vi "FlexMag - 23-03-2023.vi"() -> ()   [LabVIEW 2018] (continued)
                                }
                                }
                                }
                                }
                                }
                                }
                                }
                                }
                                frame True {
                                }
                                }
                                }
                                frame #6 {
                                n21201 = local read "abort ch3"() -> (w25287:bool)
                                n21202 = case shown="False" w25287 {
                                frame False {
                                n21203 = local read "coating start"() -> (w25288:bool)
                                n21204 = case shown="True" w25288 {
                                frame False {
                                }
                                frame True {
                                n21205 = local read "R dc step length 7"() -> (w25291:dbl)
                                n21206 = Greater?(x=w25291, y=0.0) -> (0:w25290:bool)
                                n21207 = case shown="True" w25290 {
                                frame False {
                                }
                                frame True {
                                n21208 = flat-sequence {
                                frame #0 {
                                n21209 = local read "R dc step length 7"() -> (w25298:dbl)
                                n21210 = local read "R dc step power 7"() -> (w25293:dbl)
                                n21211 = local read "R web speed"() -> (w25297:dbl)
                                n21212 = Divide(x=w25298, y=w25297) -> (x/y=w25296:dbl)
                                n21213 = Wait (ms)(milliseconds to wait=u32 100) -> ()  [unwired: 1 out]
                                n21214 = local write "Set DC Power ch2"(w25293) -> ()
                                n21215 = Multiply(x=w25296, y=60) -> (x*y=w25294:dbl)
                                n21216 = local write "time counting"(w25294) -> ()
                                }
                                frame #1 {
                                n21217 = local write "Dc_auto_set"(TRUE ("Dc_auto_set")) -> ()
                                }
                                frame #2 {
                                n21218 = while {
                                stop <- w25301 stop-if-true
                                n21219 = local read "time counting"() -> (w25307:dbl)
                                n21220 = local read "coating start"() -> (w25305:bool)
                                n21221 = local read "abort ch3"() -> (w25303:bool)
                                n21222 = Wait Until Next ms Multiple(millisecond multiple=u32 1000) -> ()  [unwired: 1 out]
                                n21223 = Decrement(x=w25307) -> (x-1=w25306:dbl)
                                n21224 = local write "time counting"(w25306) -> ()
                                n21225 = Not(x=w25305) -> (.not. x?=w25304:bool)
                                n21226 = Less Or Equal To 0?(x=w25306) -> (x <= 0?=w25302:bool)
                                n21227 = Compound Arithmetic op=OR(w25302, w25304, w25303) -> (w25301:bool)
                                }
                                }
                                }
                                }
                                }
                                }
                                }
                                }
                                frame True {
                                }
                                }
                                }
                                frame #7 {
                                n21228 = local read "abort ch3"() -> (w25308:bool)
                                n21229 = case shown="False" w25308 {
                                frame False {
                                n21230 = local read "coating start"() -> (w25309:bool)
                                n21231 = case shown="True" w25309 {
                                frame False {
                                }
                                frame True {
                                n21232 = local read "R dc step length 8"() -> (w25312:dbl)
                                n21233 = Greater?(x=w25312, y=0.0) -> (0:w25311:bool)
                                n21234 = case shown="True" w25311 {
                                frame False {
                                }
                                frame True {
                                n21235 = flat-sequence {
                                frame #0 {
                                n21236 = local read "R dc step length 8"() -> (w25319:dbl)
                                n21237 = local read "R dc step power 8"() -> (w25314:dbl)
                                n21238 = local read "R web speed"() -> (w25318:dbl)
                                n21239 = Wait (ms)(milliseconds to wait=u32 100) -> ()  [unwired: 1 out]
                                n21240 = Divide(x=w25319, y=w25318) -> (x/y=w25317:dbl)
                                n21241 = local write "Set DC Power ch2"(w25314) -> ()
                                n21242 = Multiply(x=w25317, y=60) -> (x*y=w25315:dbl)
                                n21243 = local write "time counting"(w25315) -> ()
                                }
                                frame #1 {
                                n21244 = local write "Dc_auto_set"(TRUE ("Dc_auto_set")) -> ()
                                }
                                frame #2 {
                                n21245 = while {
                                stop <- w25322 stop-if-true
                                n21246 = local read "time counting"() -> (w25328:dbl)
                                n21247 = local read "coating start"() -> (w25326:bool)
                                n21248 = Wait Until Next ms Multiple(millisecond multiple=u32 1000) -> ()  [unwired: 1 out]
                                n21249 = local read "abort ch3"() -> (w25324:bool)
                                n21250 = Decrement(x=w25328) -> (x-1=w25327:dbl)
                                n21251 = local write "time counting"(w25327) -> ()
                                n21252 = Not(x=w25326) -> (.not. x?=w25325:bool)
                                n21253 = Less Or Equal To 0?(x=w25327) -> (x <= 0?=w25323:bool)
                                n21254 = Compound Arithmetic op=OR(w25323, w25325, w25324) -> (w25322:bool)
                                }
                                }
                                }
                                }
                                }
                                }
                                }
                                }
                                frame True {
                                }
                                }
                                }
                                frame #8 {
                                n21255 = local read "abort ch3"() -> (w25329:bool)
                                n21256 = case shown="False" w25329 {
                                frame False {
                                n21257 = local read "coating start"() -> (w25330:bool)
                                n21258 = case shown="True" w25330 {
                                frame False {
                                }
                                frame True {
                                n21259 = local read "R dc step length 9"() -> (w25333:dbl)
                                n21260 = Greater?(x=w25333, y=0.0) -> (0:w25332:bool)
                                n21261 = case shown="True" w25332 {
                                frame False {
                                }
                                frame True {
                                n21262 = flat-sequence {
                                frame #0 {
                                n21263 = local read "R dc step length 9"() -> (w25340:dbl)
                                n21264 = local read "R dc step power 9"() -> (w25335:dbl)
                                n21265 = local read "R web speed"() -> (w25339:dbl)
                                n21266 = Wait (ms)(milliseconds to wait=u32 100) -> ()  [unwired: 1 out]
                                n21267 = Divide(x=w25340, y=w25339) -> (x/y=w25338:dbl)
                                n21268 = local write "Set DC Power ch2"(w25335) -> ()
                                n21269 = Multiply(x=w25338, y=60) -> (x*y=w25336:dbl)
                                n21270 = local write "time counting"(w25336) -> ()
                                }
                                frame #1 {
                                n21271 = local write "Dc_auto_set"(TRUE ("Dc_auto_set")) -> ()
                                }
                                frame #2 {
                                n21272 = while {
                                stop <- w25343 stop-if-true
                                n21273 = local read "time counting"() -> (w25349:dbl)
                                n21274 = local read "coating start"() -> (w25347:bool)
                                n21275 = local read "abort ch3"() -> (w25345:bool)
                                n21276 = Wait Until Next ms Multiple(millisecond multiple=u32 1000) -> ()  [unwired: 1 out]
                                n21277 = Decrement(x=w25349) -> (x-1=w25348:dbl)
                                n21278 = local write "time counting"(w25348) -> ()
                                n21279 = Not(x=w25347) -> (.not. x?=w25346:bool)
                                n21280 = Less Or Equal To 0?(x=w25348) -> (x <= 0?=w25344:bool)
                                n21281 = Compound Arithmetic op=OR(w25344, w25346, w25345) -> (w25343:bool)
                                }
                                }
                                }
                                }
                                }
                                }
                                }
                                }
                                frame True {
                                }
                                }
                                }
                                frame #9 {
                                n21282 = local read "abort ch3"() -> (w25350:bool)
                                n21283 = case shown="False" w25350 {
                                frame False {
                                n21284 = local read "coating start"() -> (w25351:bool)
                                n21285 = case shown="True" w25351 {
                                frame False {
                                }
                                frame True {
                                n21286 = local read "R dc step length 10"() -> (w25354:dbl)
                                n21287 = Greater?(x=w25354, y=0.0) -> (0:w25353:bool)
                                n21288 = case shown="True" w25353 {
                                frame False {
                                }
                                frame True {
                                n21289 = flat-sequence {
                                frame #0 {
                                n21290 = local read "R dc step length 10"() -> (w25361:dbl)
                                n21291 = local read "R dc step power 10"() -> (w25356:dbl)
                                n21292 = local read "R web speed"() -> (w25360:dbl)
                                n21293 = Divide(x=w25361, y=w25360) -> (x/y=w25359:dbl)
                                n21294 = local write "Set DC Power ch2"(w25356) -> ()
                                n21295 = Wait (ms)(milliseconds to wait=u32 100) -> ()  [unwired: 1 out]
                                n21296 = Multiply(x=w25359, y=60) -> (x*y=w25357:dbl)
                                n21297 = local write "time counting"(w25357) -> ()
                                }
                                frame #1 {
                                n21298 = local write "Dc_auto_set"(TRUE ("Dc_auto_set")) -> ()
                                }
                                frame #2 {
                                n21299 = while {
                                stop <- w25364 stop-if-true
                                n21300 = local read "time counting"() -> (w25370:dbl)
                                n21301 = local read "coating start"() -> (w25368:bool)
                                n21302 = local read "abort ch3"() -> (w25366:bool)
                                n21303 = Wait Until Next ms Multiple(millisecond multiple=u32 1000) -> ()  [unwired: 1 out]
                                n21304 = Decrement(x=w25370) -> (x-1=w25369:dbl)
                                n21305 = local write "time counting"(w25369) -> ()
                                n21306 = Not(x=w25368) -> (.not. x?=w25367:bool)
                                n21307 = Less Or Equal To 0?(x=w25369) -> (x <= 0?=w25365:bool)
                                n21308 = Compound Arithmetic op=OR(w25365, w25367, w25366) -> (w25364:bool)
                                }
                                }
                                }
                                }
                                }
                                }
                                }
                                }
                                frame True {
                                }
                                }
                                }
                                frame #10 {
                                n21309 = local read "abort ch3"() -> (w25371:bool)
                                n21310 = case shown="False" w25371 {
                                frame False {
                                n21311 = local read "coating start"() -> (w25372:bool)
                                n21312 = case shown="True" w25372 {
                                frame False {
                                }
                                frame True {
                                n21313 = Wait (ms)(milliseconds to wait=u32 100) -> ()  [unwired: 1 out]
                                "coating ch3 led 12" <- TRUE ("coating ch2 led 1")
                                }
                                }
                                }
                                frame True {
                                }
                                }
                                }
                                }
                                }
                                frame Enabled {
                                n21314 = stacked-sequence {
                                frame #0 {
                                n21315 = local read "abort ch3"() -> (w25375:bool)
                                n21316 = case shown="False" w25375 {
                                frame False {
                                n21317 = local read "coating start"() -> (w25376:bool)
                                n21318 = case shown="True" w25376 {
                                frame False {
                                }
                                frame True {
                                n21319 = local read "dep. for?"() -> (w25377:bool)
                                n21320 = case shown="False" w25377 {
                                frame False {
                                n21321 = flat-sequence {
                                frame #0 {
                                n21322 = local read "R DC number steps"() -> (w25380:dbl)
                                n21323 = case shown="20" w25380 {
                                tunnel: [0.0 ("step up") 1.0 ("step up") 2.0 ("step up") 3.0 ("step up") 4.0 ("step up") 5.0 ("step up") 6.0 ("step up") 7.0 ("step up") 8.0 ("step up") 9.0 ("step up") 10.0 ("step up") 11.0 ("step up") 12.0 ("step up") 13.0 ("step up") 14.0 ("step up") 15.0 ("step up") 16.0 ("step up") 17.0 ("step up") 18.0 ("step up") 19.0 ("step up") 20.0 ("step up")] -> w25379
                                tunnel: [200.0 ("R dc step power 1") w25385 w25387 w25389 w25391 w25393 w25395 w25397 w25399 w25401 w25403 w25405 w25407 w25409 w25411 w25413 w25415 w25417 w25419 w25421 w25423] -> w25378
                                frame 0, Default {
                                }
                                frame 1 {
                                n21324 = local read "R dc step power 1"() -> (w25385:dbl)
                                }
                                frame 2 {
                                n21325 = local read "R dc step power 2"() -> (w25387:dbl)
                                }
                                frame 3 {
                                n21326 = local read "R dc step power 3"() -> (w25389:dbl)
                                }
                                frame 4 {
                                n21327 = local read "R dc step power 4"() -> (w25391:dbl)
                                }
                                frame 5 {
                                n21328 = local read "R dc step power 5"() -> (w25393:dbl)
                                }
                                frame 6 {
                                n21329 = local read "R dc step power 6"() -> (w25395:dbl)
                                }
                                frame 7 {
                                n21330 = local read "R dc step power 7"() -> (w25397:dbl)
                                }
                                frame 8 {
                                n21331 = local read "R dc step power 8"() -> (w25399:dbl)
                                }
                                frame 9 {
                                n21332 = local read "R dc step power 9"() -> (w25401:dbl)
                                }
                                frame 10 {
                                n21333 = local read "R dc step power 10"() -> (w25403:dbl)
                                }
                                frame 11 {
                                n21334 = local read "R dc step power 11"() -> (w25405:dbl)
                                }
                                frame 12 {
                                n21335 = local read "R dc step power 12"() -> (w25407:dbl)
                                }
                                frame 13 {
                                n21336 = local read "R dc step power 13"() -> (w25409:dbl)
                                }
                                frame 14 {
                                n21337 = local read "R dc step power 14"() -> (w25411:dbl)
                                }
                                frame 15 {
                                n21338 = local read "R dc step power 15"() -> (w25413:dbl)
                                }
                                frame 16 {
                                n21339 = local read "R dc step power 16"() -> (w25415:dbl)
                                }
                                frame 17 {
                                n21340 = local read "R dc step power 17"() -> (w25417:dbl)
                                }
                                frame 18 {
                                n21341 = local read "R dc step power 18"() -> (w25419:dbl)
                                }
                                frame 19 {
                                n21342 = local read "R dc step power 19"() -> (w25421:dbl)
                                }
                                frame 20 {
                                n21343 = local read "R dc step power 20"() -> (w25423:dbl)
                                }
                                }
                                n21344 = Wait (ms)(milliseconds to wait=u32 100) -> ()  [unwired: 1 out]
                                n21345 = local write "current step"(w25379) -> ()
                                n21346 = local write "Set DC Power auto"(w25378) -> ()
                                }
                                frame #1 {
                                n21347 = local write "Dc_auto_set"(TRUE ("Dc_auto_set")) -> ()
                                }
                                frame #2 {
                                n21348 = Wait (ms)(milliseconds to wait=u32 1000) -> ()  [unwired: 1 out]
                                }
                                }
                                }
                                frame True {
                                n21349 = flat-sequence {
                                frame #0 {
                                n21350 = local read "R dc step power 1"() -> (w25428:dbl)
                                n21351 = Wait (ms)(milliseconds to wait=u32 100) -> ()  [unwired: 1 out]
                                n21352 = local write "Set DC Power auto"(w25428) -> ()
                                n21353 = local write "current step"(1.0 ("step up")) -> ()
                                }
                                frame #1 {
                                n21354 = local write "Dc_auto_set"(TRUE ("Dc_auto_set")) -> ()
                                }
                                frame #2 {
                                n21355 = Wait (ms)(milliseconds to wait=u32 1000) -> ()  [unwired: 1 out]
                                }
                                }
                                }
                                }
                                }
                                }
                                }
                                frame True {
                                }
                                }
                                }
                                frame #1 {
                                n21356 = local read "abort ch3"() -> (w25431:bool)
                                n21357 = case shown="False" w25431 {
                                frame False {
                                n21358 = local read "coating start"() -> (w25432:bool)
                                n21359 = case shown="True" w25432 {
                                frame False {
                                }
                                frame True {
                                n21360 = while {
                                i -> [w25441]
                                stop <- w25445 stop-if-true
                                n21361 = local read "roll error (min)"() -> (w25434:i32)
                                n21362 = local read "step count"() -> (w25448:dbl)
                                n21363 = local read "R DC number steps"() -> (w25446:dbl)
                                n21364 = Multiply(x=200, y=w25434) -> (x*y=w25435:i32)
                                n21365 = feedback #341() -> (w25449:dbl)  [unwired: 1 in]
                                n21366 = feedback-in #341(w25448) -> ()
                                n21367 = Wait Until Next ms Multiple(millisecond multiple=u32 300) -> ()  [unwired: 1 out]
                                n21368 = Greater?(x=w25441, y=w25435) -> (0:w25433:bool)
                                n21369 = Less?(x=w25448, y=w25449) -> (x < y?=w25447:bool)
                                n21370 = case shown="True" w25433 {
                                frame False {
                                }
                                frame True {
                                n21371 = local write "Warning Message"("Automatic Coating Process is canceled !\nCH3  rolling problem..." ("Warning Message")) -> ()
                                n21372 = local write "coating error"(TRUE ("coating error")) -> ()
                                }
                                }
                                n21373 = case shown="True" w25447 {
                                tunnel: w25446 -> [_ w25456]
                                tunnel: [FALSE w25454] -> w25443
                                frame False {
                                }
                                frame True {
                                n21374 = local read "current step"() -> (w25455:dbl)
                                n21375 = Greater Or Equal?(x=w25456, y=w25455) -> (x >= y?=w25453:bool)
                                n21376 = Not(x=w25453) -> (.not. x?=w25454:bool)
                                n21377 = case shown="True" w25453 {
                                tunnel: w25455 -> [_ w25457]
                                frame False {
                                }
                                frame True {
                                n21378 = case shown="10" w25457 {
                                frame 0, Default {
                                }
                                frame 1 {
                                n21379 = stacked-sequence {
                                frame #0 {
                                n21380 = local read "R dc step power 1"() -> (w25459:dbl)
                                n21381 = local write "Set DC Power auto"(w25459) -> ()
                                n21382 = Wait (ms)(milliseconds to wait=u32 100) -> ()  [unwired: 1 out]
                                }
                                frame #1 {
                                n21383 = local write "Dc_auto_set"(TRUE ("Dc_auto_set")) -> ()
                                }
                                }
                                }
                                frame 2 {
                                n21384 = stacked-sequence {
                                frame #0 {
                                n21385 = local read "R dc step power 2"() -> (w25462:dbl)
                                n21386 = local write "Set DC Power auto"(w25462) -> ()
                                n21387 = Wait (ms)(milliseconds to wait=u32 100) -> ()  [unwired: 1 out]
                                }
                                frame #1 {
                                n21388 = local write "Dc_auto_set"(TRUE ("Dc_auto_set")) -> ()
                                }
                                }
                                }
                                frame 3 {
                                n21389 = stacked-sequence {
                                frame #0 {
                                n21390 = local read "R dc step power 3"() -> (w25465:dbl)
                                n21391 = local write "Set DC Power auto"(w25465) -> ()
                                n21392 = Wait (ms)(milliseconds to wait=u32 100) -> ()  [unwired: 1 out]
                                }
                                frame #1 {
                                n21393 = local write "Dc_auto_set"(TRUE ("Dc_auto_set")) -> ()
                                }
                                }
                                }
                                frame 4 {
                                n21394 = stacked-sequence {
                                frame #0 {
                                n21395 = local read "R dc step power 4"() -> (w25468:dbl)
                                n21396 = local write "Set DC Power auto"(w25468) -> ()
                                n21397 = Wait (ms)(milliseconds to wait=u32 100) -> ()  [unwired: 1 out]
                                }
                                frame #1 {
                                n21398 = local write "Dc_auto_set"(TRUE ("Dc_auto_set")) -> ()
                                }
                                }
                                }
                                frame 5 {
                                n21399 = stacked-sequence {
                                frame #0 {
                                n21400 = local read "R dc step power 5"() -> (w25471:dbl)
                                n21401 = local write "Set DC Power auto"(w25471) -> ()
                                n21402 = Wait (ms)(milliseconds to wait=u32 100) -> ()  [unwired: 1 out]
                                }
                                frame #1 {
                                n21403 = local write "Dc_auto_set"(TRUE ("Dc_auto_set")) -> ()
                                }
                                }
                                }
                                frame 6 {
                                n21404 = stacked-sequence {
                                frame #0 {
                                n21405 = local read "R dc step power 6"() -> (w25474:dbl)
                                n21406 = local write "Set DC Power auto"(w25474) -> ()
                                n21407 = Wait (ms)(milliseconds to wait=u32 100) -> ()  [unwired: 1 out]
                                }
                                frame #1 {
                                n21408 = local write "Dc_auto_set"(TRUE ("Dc_auto_set")) -> ()
                                }
                                }
                                }
                                frame 7 {
                                n21409 = stacked-sequence {
                                frame #0 {
                                n21410 = local read "R dc step power 7"() -> (w25477:dbl)
                                n21411 = local write "Set DC Power auto"(w25477) -> ()
                                n21412 = Wait (ms)(milliseconds to wait=u32 100) -> ()  [unwired: 1 out]
                                }
                                frame #1 {
                                n21413 = local write "Dc_auto_set"(TRUE ("Dc_auto_set")) -> ()
                                }
                                }
                                }
                                frame 8 {
                                n21414 = stacked-sequence {
                                frame #0 {
                                n21415 = local read "R dc step power 8"() -> (w25480:dbl)
                                n21416 = local write "Set DC Power auto"(w25480) -> ()
                                n21417 = Wait (ms)(milliseconds to wait=u32 100) -> ()  [unwired: 1 out]
                                }
                                frame #1 {
                                n21418 = local write "Dc_auto_set"(TRUE ("Dc_auto_set")) -> ()
                                }
                                }
                                }
                                frame 9 {
                                n21419 = stacked-sequence {
                                frame #0 {
                                n21420 = local read "R dc step power 9"() -> (w25483:dbl)
                                n21421 = local write "Set DC Power auto"(w25483) -> ()
                                n21422 = Wait (ms)(milliseconds to wait=u32 100) -> ()  [unwired: 1 out]
                                }
                                frame #1 {
                                n21423 = local write "Dc_auto_set"(TRUE ("Dc_auto_set")) -> ()
                                }
                                }
                                }
                                frame 10 {
                                n21424 = stacked-sequence {
                                frame #0 {
                                n21425 = local read "R dc step power 10"() -> (w25486:dbl)
                                n21426 = local write "Set DC Power auto"(w25486) -> ()
                                n21427 = Wait (ms)(milliseconds to wait=u32 100) -> ()  [unwired: 1 out]
                                }
                                frame #1 {
                                n21428 = local write "Dc_auto_set"(TRUE ("Dc_auto_set")) -> ()
                                }
                                }
                                }
                                frame 11 {
                                n21429 = stacked-sequence {
                                frame #0 {
                                n21430 = local read "R dc step power 11"() -> (w25489:dbl)
                                n21431 = local write "Set DC Power auto"(w25489) -> ()
                                n21432 = Wait (ms)(milliseconds to wait=u32 100) -> ()  [unwired: 1 out]
                                }
                                frame #1 {
                                n21433 = local write "Dc_auto_set"(TRUE ("Dc_auto_set")) -> ()
                                }
                                }
                                }
                                frame 12 {
                                n21434 = stacked-sequence {
                                frame #0 {
                                n21435 = local read "R dc step power 12"() -> (w25492:dbl)
                                n21436 = local write "Set DC Power auto"(w25492) -> ()
                                n21437 = Wait (ms)(milliseconds to wait=u32 100) -> ()  [unwired: 1 out]
                                }
                                frame #1 {
                                n21438 = local write "Dc_auto_set"(TRUE ("Dc_auto_set")) -> ()
                                }
                                }
                                }
                                frame 13 {
                                n21439 = stacked-sequence {
                                frame #0 {
                                n21440 = local read "R dc step power 13"() -> (w25495:dbl)
                                n21441 = local write "Set DC Power auto"(w25495) -> ()
                                n21442 = Wait (ms)(milliseconds to wait=u32 100) -> ()  [unwired: 1 out]
                                }
                                frame #1 {
                                n21443 = local write "Dc_auto_set"(TRUE ("Dc_auto_set")) -> ()
                                }
                                }
                                }
                                frame 14 {
                                n21444 = stacked-sequence {
                                frame #0 {
                                n21445 = local read "R dc step power 14"() -> (w25498:dbl)
                                n21446 = local write "Set DC Power auto"(w25498) -> ()
                                n21447 = Wait (ms)(milliseconds to wait=u32 100) -> ()  [unwired: 1 out]
                                }
                                frame #1 {
                                n21448 = local write "Dc_auto_set"(TRUE ("Dc_auto_set")) -> ()
                                }
                                }
                                }
                                frame 15 {
                                n21449 = stacked-sequence {
                                frame #0 {
                                n21450 = local read "R dc step power 15"() -> (w25501:dbl)
                                n21451 = local write "Set DC Power auto"(w25501) -> ()
                                n21452 = Wait (ms)(milliseconds to wait=u32 100) -> ()  [unwired: 1 out]
                                }
                                frame #1 {
                                n21453 = local write "Dc_auto_set"(TRUE ("Dc_auto_set")) -> ()
                                }
                                }
                                }
                                frame 16 {
                                n21454 = stacked-sequence {
                                frame #0 {
                                n21455 = local read "R dc step power 16"() -> (w25504:dbl)
                                n21456 = local write "Set DC Power auto"(w25504) -> ()
                                n21457 = Wait (ms)(milliseconds to wait=u32 100) -> ()  [unwired: 1 out]
                                }
                                frame #1 {
                                n21458 = local write "Dc_auto_set"(TRUE ("Dc_auto_set")) -> ()
                                }
                                }
                                }
                                frame 17 {
                                n21459 = stacked-sequence {
                                frame #0 {
                                n21460 = local read "R dc step power 17"() -> (w25507:dbl)
                                n21461 = local write "Set DC Power auto"(w25507) -> ()
                                n21462 = Wait (ms)(milliseconds to wait=u32 100) -> ()  [unwired: 1 out]
                                }
                                frame #1 {
                                n21463 = local write "Dc_auto_set"(TRUE ("Dc_auto_set")) -> ()
                                }
                                }
                                }
                                frame 18 {
                                n21464 = stacked-sequence {
                                frame #0 {
                                n21465 = local read "R dc step power 18"() -> (w25510:dbl)
                                n21466 = local write "Set DC Power auto"(w25510) -> ()
                                n21467 = Wait (ms)(milliseconds to wait=u32 100) -> ()  [unwired: 1 out]
                                }
                                frame #1 {
                                n21468 = local write "Dc_auto_set"(TRUE ("Dc_auto_set")) -> ()
                                }
                                }
                                }
                                frame 19 {
                                n21469 = stacked-sequence {
                                frame #0 {
                                n21470 = local read "R dc step power 19"() -> (w25513:dbl)
                                n21471 = local write "Set DC Power auto"(w25513) -> ()
                                n21472 = Wait (ms)(milliseconds to wait=u32 100) -> ()  [unwired: 1 out]
                                }
                                frame #1 {
                                n21473 = local write "Dc_auto_set"(TRUE ("Dc_auto_set")) -> ()
                                }
                                }
                                }
                                frame 20 {
                                n21474 = stacked-sequence {
                                frame #0 {
                                n21475 = local read "R dc step power 20"() -> (w25516:dbl)
                                n21476 = local write "Set DC Power auto"(w25516) -> ()
                                n21477 = Wait (ms)(milliseconds to wait=u32 100) -> ()  [unwired: 1 out]
                                }
                                frame #1 {
                                n21478 = local write "Dc_auto_set"(TRUE ("Dc_auto_set")) -> ()
                                }
                                }
                                }
                                }
                                }
                                }
                                }
                                }
                                n21479 = local read "CH3_Motor DO"() -> (w25438:bool)
                                n21480 = local read "coating start"() -> (w25444:bool)
                                n21481 = local read "abort ch3"() -> (w25440:bool)
                                n21482 = Not(x=w25444) -> (.not. x?=w25439:bool)
                                n21483 = Not(x=w25438) -> (.not. x?=w25437:bool)
                                n21484 = Compound Arithmetic op=OR(w25443, w25440, w25439, w25437) -> (w25445:bool)
                                }
                                }
                                }
                                }
                                frame True {
                                }
                                }
                                }
                                }
                                }
                                }
                                }
                                frame #13 {
                                # "DC off"
                                n21485 = stacked-sequence {
                                frame #0 {
                                n21486 = local read "abort ch3"() -> (w25518:bool)
                                n21487 = case shown="False" w25518 {
                                frame False {
                                n21488 = local read "coating start"() -> (w25519:bool)
                                n21489 = case shown="True" w25519 {
                                frame False {
                                }
                                frame True {
                                n21490 = stacked-sequence {
                                frame #0 {
                                n21491 = Wait (ms)(milliseconds to wait=u32 1000) -> ()  [unwired: 1 out]
                                }
                                frame #1 {
                                n21492 = flat-sequence {
                                frame #0 {
                                n21493 = local write "Dc_auto_off"(TRUE ("Dc_auto_off")) -> ()
                                }
                                frame #1 {
                                n21494 = local write "Set DC Power auto"(0.0 ("Set DC Power")) -> ()
                                n21495 = local write "Dc_auto_off"(FALSE ("Dc_auto_off")) -> ()
                                n21496 = Wait (ms)(milliseconds to wait=u32 3000) -> ()  [unwired: 1 out]
                                }
                                frame #2 {
                                n21497 = local write "Dc_auto_off"(TRUE ("Dc_auto_off")) -> ()
                                }
                                frame #3 {
                                n21498 = Wait (ms)(milliseconds to wait=u32 1000) -> ()  [unwired: 1 out]
                                }
                                }
                                }
                                }
                                }
                                }
                                }
                                frame True {
                                }
                                }
                                }
                                frame #1 {
                                n21499 = local read "abort ch3"() -> (w25527:bool)
                                n21500 = case shown="False" w25527 {
                                frame False {
                                n21501 = local read "coating start"() -> (w25528:bool)
                                n21502 = case shown="True" w25528 {
                                frame False {
                                }
                                frame True {
                                n21503 = while {
                                i -> [w25531]
                                stop <- w25533 stop-if-true
                                n21504 = Greater Or Equal?(x=w25531, y=10) -> (x >= y?=w25532:bool)
                                n21505 = case shown="True" w25532 {
                                frame False {
                                }
                                frame True {
                                n21506 = local write "Warning Message"("Automatic Coating Process is canceled !\nDCPS cannot be turned off." ("Warning Message")) -> ()
                                n21507 = local write "coating error"(TRUE ("coating error")) -> ()
                                }
                                }
                                n21508 = local read "Dcps_is_on"() -> (w25537:bool)
                                n21509 = case shown="True" w25537 {
                                tunnel: [TRUE ("CH2_WFC_DO") FALSE ("CH2_WFC_DO")] -> w25536
                                frame False {
                                }
                                frame True {
                                n21510 = Wait Until Next ms Multiple(millisecond multiple=u32 1000) -> ()  [unwired: 1 out]
                                n21511 = local write "Dc_auto_off"(TRUE ("coating error")) -> ()
                                }
                                }
                                n21512 = local read "coating start"() -> (w25535:bool)
                                n21513 = local read "abort ch3"() -> (w25529:bool)
                                n21514 = Not(x=w25535) -> (.not. x?=w25534:bool)
                                n21515 = Compound Arithmetic op=OR(w25536, w25534, w25529) -> (w25533:bool)
                                }
                                }
                                }
                                }
                                frame True {
                                }
                                }
                                }
                                frame #2 {
                                n21516 = local read "abort ch3"() -> (w25544:bool)
                                n21517 = case shown="False" w25544 {
                                frame False {
                                n21518 = local read "coating start"() -> (w25545:bool)
                                n21519 = case shown="True" w25545 {
                                frame False {
                                }
                                frame True {
                                n21520 = Wait (ms)(milliseconds to wait=u32 100) -> ()  [unwired: 1 out]
                                "coating ch3 led 13" <- TRUE ("coating ch2 led 1")
                                }
                                }
                                }
                                frame True {
                                }
                                }
                                }
                                }
                                }
                                frame #14 {
                                # "pcgv open"
                                n21521 = stacked-sequence {
                                frame #0 {
                                n21522 = local read "abort ch3"() -> (w25548:bool)
                                n21523 = case shown="False" w25548 {
                                frame False {
                                n21524 = local read "coating start"() -> (w25549:bool)
                                n21525 = case shown="True" w25549 {
                                frame False {
                                }
                                frame True {
                                n21526 = local write "pcgv3 auto open"(TRUE ("ch3 ar set zero auto")) -> ()
                                }
                                }
                                }
                                frame True {
                                }
                                }
                                }
                                frame #1 {
                                n21527 = local read "abort ch3"() -> (w25551:bool)
                                n21528 = case shown="False" w25551 {
                                frame False {
                                n21529 = local read "coating start"() -> (w25552:bool)
                                n21530 = case shown="True" w25552 {
                                frame False {
                                }
                                frame True {
                                n21531 = while {
                                i -> [w25556]
                                stop <- w25558 stop-if-true
                                n21532 = Greater Or Equal?(x=w25556, y=50) -> (x >= y?=w25557:bool)
                                n21533 = case shown="True" w25557 {
                                frame False {
                                }
                                frame True {
                                n21534 = local write "Warning Message"("Automatic Coating Process is canceled !\nCH3 PCGV couldn't be opened..." ("Warning Message")) -> ()
                                n21535 = local write "coating error"(TRUE ("coating error")) -> ()
                                }
                                }
                                n21536 = local read "ch3_pcgv_gui"() -> (w25553:bool)
                                n21537 = case shown="False" w25553 {
                                tunnel: [FALSE ("CH2_WFC_DO") TRUE ("CH2_WFC_DO")] -> w25561
                                frame False {
                                n21538 = Wait Until Next ms Multiple(millisecond multiple=u32 1000) -> ()  [unwired: 1 out]
                                n21539 = local write "pcgv3 auto open"(TRUE ("coating error")) -> ()
                                }
                                frame True {
                                }
                                }
                                n21540 = local read "coating start"() -> (w25560:bool)
                                n21541 = local read "abort ch3"() -> (w25554:bool)
                                n21542 = Not(x=w25560) -> (.not. x?=w25559:bool)
                                n21543 = Compound Arithmetic op=OR(w25561, w25559, w25554) -> (w25558:bool)
                                }
                                }
                                }
                                }
                                frame True {
                                }
                                }
                                }
                                frame #2 {
                                n21544 = local read "abort ch3"() -> (w25568:bool)
                                n21545 = case shown="False" w25568 {
                                frame False {
                                n21546 = local read "coating start"() -> (w25569:bool)
                                n21547 = case shown="True" w25569 {
                                frame False {
                                }
                                frame True {
                                n21548 = Wait (ms)(milliseconds to wait=u32 100) -> ()  [unwired: 1 out]
                                "coating ch3 led 14" <- TRUE ("coating ch2 led 1")
                                }
                                }
                                }
                                frame True {
                                }
                                }
                                }
                                }
                                }
                                frame #15 {
                                # "argon set zero"
                                n21549 = stacked-sequence {
                                frame #0 {
                                n21550 = local read "abort ch3"() -> (w25572:bool)
                                n21551 = case shown="False" w25572 {
                                frame False {
                                n21552 = local read "coating start"() -> (w25573:bool)
                                n21553 = case shown="True" w25573 {
                                frame False {
                                }
                                frame True {
                                n21554 = local write "ch3 ar set zero auto"(TRUE ("ch3 ar set zero auto")) -> ()
                                }
                                }
                                }
                                frame True {
                                }
                                }
                                }
                                frame #1 {
                                n21555 = local read "abort ch3"() -> (w25575:bool)
                                n21556 = case shown="False" w25575 {
                                frame False {
                                n21557 = local read "coating start"() -> (w25576:bool)
                                n21558 = case shown="True" w25576 {
                                frame False {
                                }
                                frame True {
                                n21559 = while {
                                i -> [w25582]
                                stop <- w25584 stop-if-true
                                n21560 = Greater Or Equal?(x=w25582, y=50) -> (x >= y?=w25583:bool)
                                n21561 = case shown="True" w25583 {
                                frame False {
                                }
                                frame True {
                                n21562 = local write "Warning Message"("Automatic Coating Process is canceled !\nCH3 Argon Set Zero problem..." ("Warning Message")) -> ()
                                n21563 = local write "coating error"(TRUE ("coating error")) -> ()
                                }
                                }
                                n21564 = local read "ch3 argon mfc actual"() -> (w25578:dbl)
                                n21565 = Less?(x=w25578, y=1.0) -> (x < y?=w25579:bool)
                                n21566 = case shown="False" w25579 {
                                tunnel: [FALSE ("CH2_WFC_DO") TRUE ("CH2_WFC_DO")] -> w25587
                                frame False {
                                n21567 = Wait Until Next ms Multiple(millisecond multiple=u32 1000) -> ()  [unwired: 1 out]
                                n21568 = local write "ch3 ar set zero auto"(TRUE ("coating error")) -> ()
                                }
                                frame True {
                                }
                                }
                                n21569 = local read "coating start"() -> (w25586:bool)
                                n21570 = local read "abort ch3"() -> (w25580:bool)
                                n21571 = Not(x=w25586) -> (.not. x?=w25585:bool)
                                n21572 = Compound Arithmetic op=OR(w25587, w25585, w25580) -> (w25584:bool)
                                }
                                }
                                }
                                }
                                frame True {
                                }
                                }
                                }
                                frame #2 {
                                n21573 = local read "abort ch3"() -> (w25594:bool)
                                n21574 = case shown="False" w25594 {
                                frame False {
                                n21575 = local read "coating start"() -> (w25595:bool)
                                n21576 = case shown="True" w25595 {
                                frame False {
                                }
                                frame True {
                                n21577 = Wait (ms)(milliseconds to wait=u32 100) -> ()  [unwired: 1 out]
                                "coating ch3 led 15" <- TRUE ("coating ch2 led 1")
                                }
                                }
                                }
                                frame True {
                                }
                                }
                                }
                                }
                                }
                                frame #16 {
                                # "Ar SoV close"
                                n21578 = stacked-sequence {
                                frame #0 {
                                n21579 = local read "abort ch3"() -> (w25598:bool)
                                n21580 = case shown="False" w25598 {
                                frame False {
                                n21581 = local read "coating start"() -> (w25599:bool)
                                n21582 = case shown="True" w25599 {
                                frame False {
                                }
                                frame True {
                                n21583 = while {
                                i -> [w25603]
                                stop <- w25605 stop-if-true
                                n21584 = Greater Or Equal?(x=w25603, y=100) -> (x >= y?=w25604:bool)
                                n21585 = case shown="True" w25604 {
                                frame False {
                                }
                                frame True {
                                n21586 = local write "Warning Message"("Automatic Coating Process is canceled !\nCH3 Argon SoV couldn't be closed..." ("Warning Message")) -> ()
                                n21587 = local write "coating error"(TRUE ("coating error")) -> ()
                                }
                                }
                                n21588 = local read "CH3_SoV_Ar_DI"() -> (w25600:bool)
                                n21589 = case shown="True" w25600 {
                                tunnel: [TRUE ("CH2_WFC_DO") FALSE ("CH2_WFC_DO")] -> w25608
                                frame False {
                                }